vi "ATF_PUMP_PID_screen_V0.1.vi"() -> ()   [LabVIEW 2022 SP3]
panel:
  out "Countdown Timer (CDT)":dbl format="T%<+%H:%M:%S%3u>t"
  out "Date":timestamp format="%<%d/%m/%Y>T"
  in  "Close":bool
  in  "Screen No":dbl
  out "Indian Standard Time (IST)":timestamp format="%<%H:%M:%S%2u>T"
  out "B_AT_T_04 27":dbl format="%.2f bar"
  out "B_AT_T_04 26":dbl format="%.2f bar"
  out "B_AT_T_04 25":dbl format="%.2f bar"
  out "B_AT_T_04 21":dbl format="%.2f bar"
  out "B_AT_T_04":dbl format="%.2f bar"
  out "B_AT_T_05":dbl format="%.2f bar"
  out "B_LO_P_09":dbl format="%.2f bar"
  out "B_LO_P_10":dbl format="%.2f bar"
  out "B_AT_T_05":dbl format="%.2f bar"
  out "B_AT_T_04":dbl format="%.2f bar"
  out "B_LO_P_10":dbl format="%.2f bar"
  out "B_LO_P_09":dbl format="%.2f bar"
  # "BSTF P&ID SCREEN"
  # "VERSION 1.0"
  # "ATF MANIFOLD"
  # "ATF MANIFOLD"
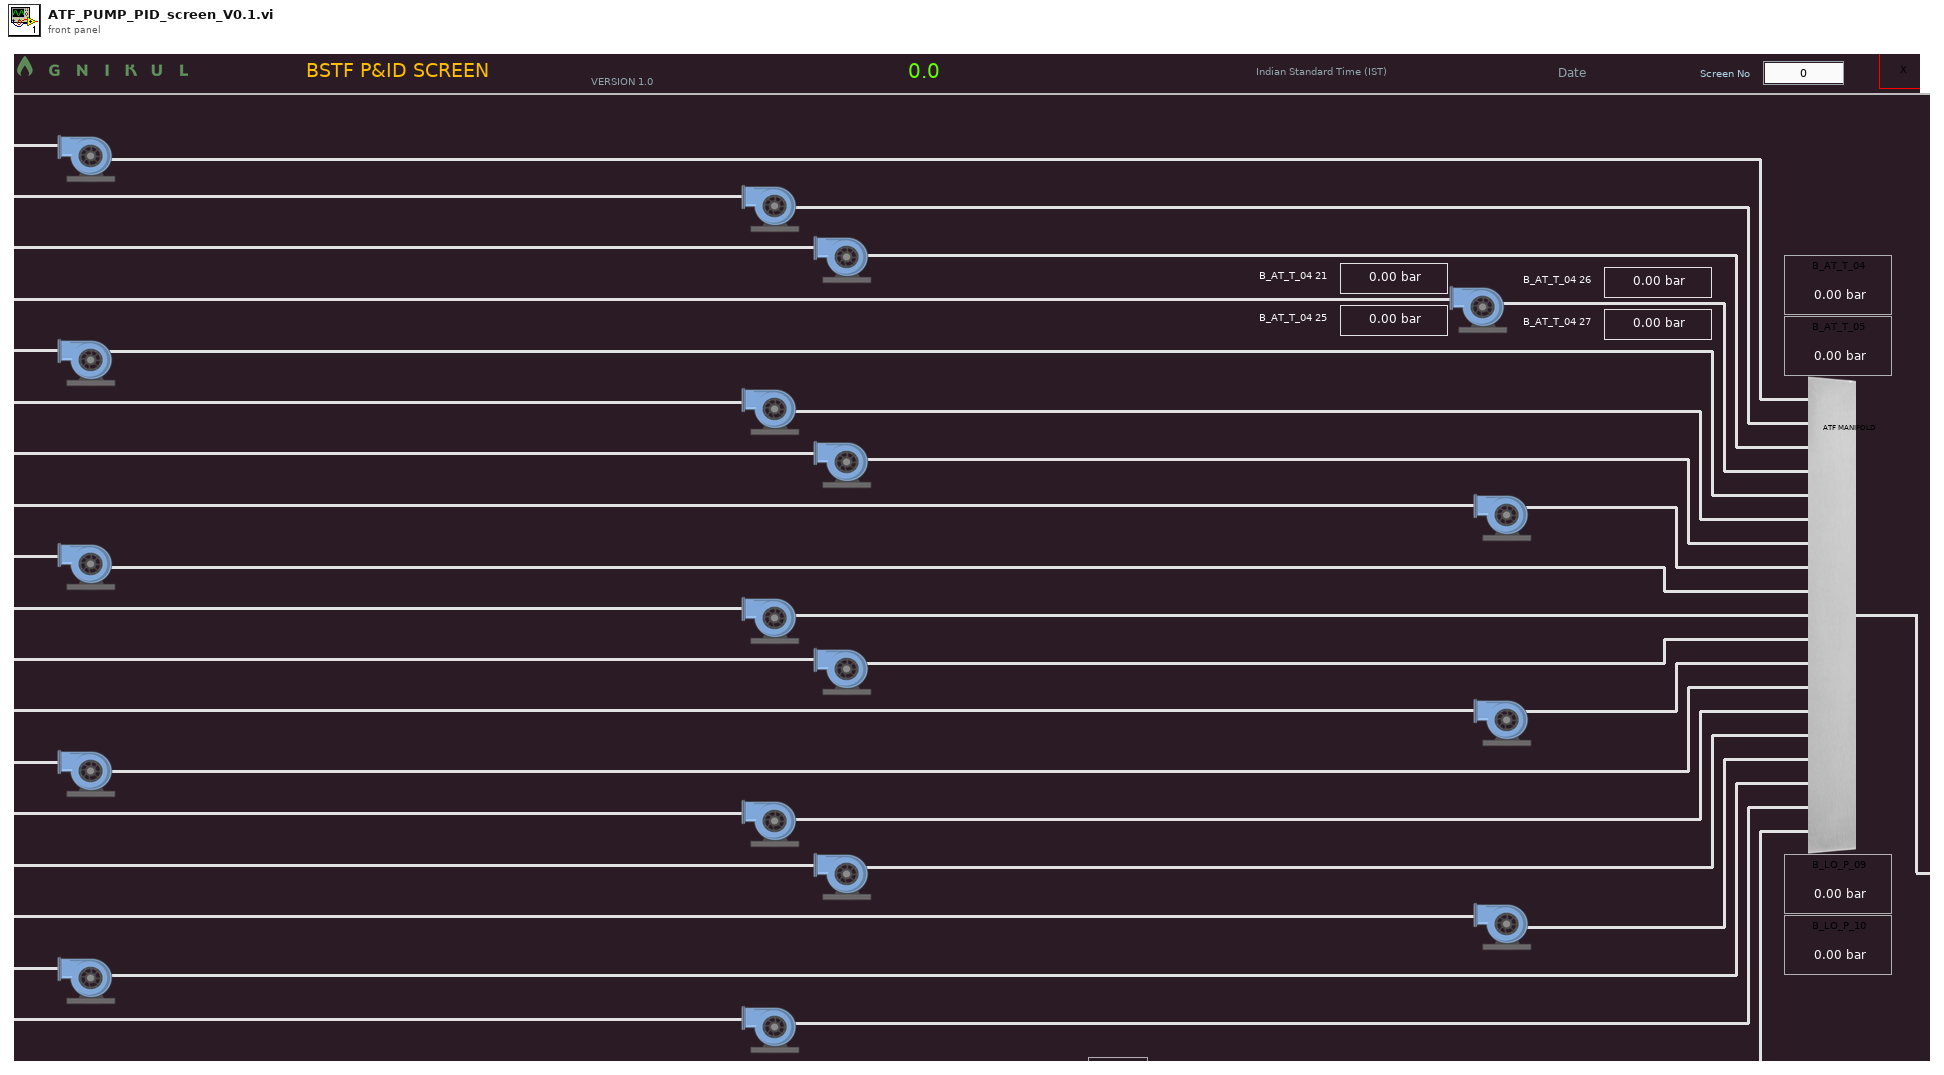
[diagram p1: front panel]
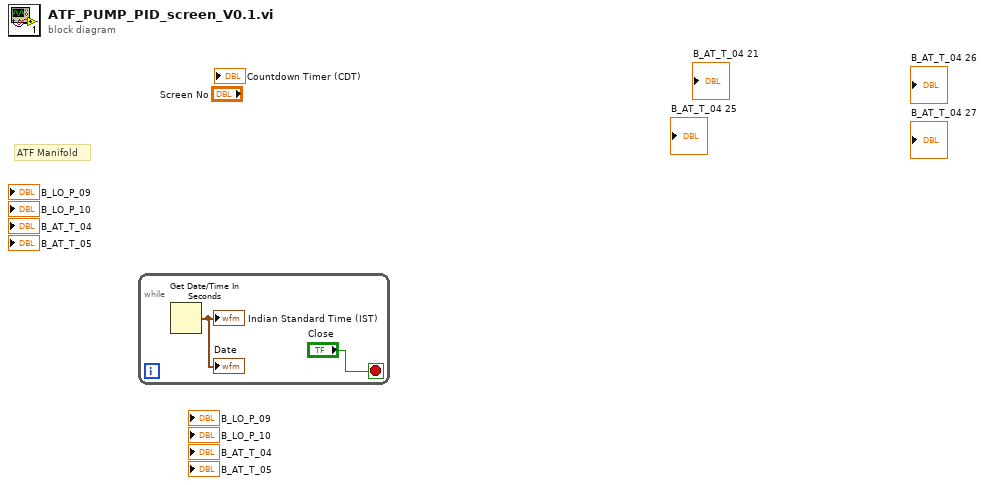
[diagram p0: block diagram]
diagram:
  # "ATF Manifold"
  n1 = while {
    stop <- "Close" stop-if-true
    n2 = Get Date/Time In Seconds() -> (seconds since 1Jan1904=→"Date" →"Indian Standard Time (IST)":timestamp)
  }
